vi "HFRR ADV v038.vi"() -> ()   [LabVIEW 2025] (continued)
              }
              frame #2 {
                n259 = local write "Due Write"("VC;0") -> ()
              }
              frame #3 {
                n260 = Wait (ms)(milliseconds to wait=u32 2000) -> ()  [unwired: 1 out]
              }
              frame #4 {
                w347 = T19."Enabled" ("Disabled")
                (unwired) T26."Imaging" ("Main Dashboard Buttons")
                w348 = "" ("FILE")
                n261 = local write "Main Tab"(T2."Adv Scar" ("Main Tab")) -> ()
                n262 = local write "measured_stroke"(0.0 ("measured_stroke")) -> ()
                n263 = local write "Main Dashboard Buttons"(T1."Imaging" ("Main Dashboard Buttons")) -> ()
                n264 = property on="RUN" class="Bool (strict)"("Visible"=TRUE) -> ()  [unwired: 2 in, 2 out]
                n265 = local write "Due Write"("VC;0") -> ()
                n266 = local write "Humidity"(TRUE ("Humidity")) -> ()
                n267 = local write "TEST FILE NAM,E SAVED"(FALSE ("TEST FILE NAM,E SAVED")) -> ()
                n268 = local write "Fuel Discription :"(w348) -> ()
                n269 = local write "Batch Ref Num :"(w348) -> ()
                n270 = local write "Remarks :"(w348) -> ()
                n271 = local write "FILE"(w348) -> ()
                n272 = property on="FRICVALZ 2" class="Bool (strict)"("DisabledEnum"=w347) -> ()  [unwired: 2 in, 2 out]
                n273 = property on="FRICVALZ 4" class="Bool (strict)"("DisabledEnum"=w347) -> ()  [unwired: 2 in, 2 out]
                n274 = property on="FRICVALZ 3" class="Bool (strict)"("DisabledEnum"=w347) -> ()  [unwired: 2 in, 2 out]
              }
            }
          }
          frame True {
            n275 = stacked-sequence {
              frame #0 {
                n276 = local write "Due Write"("DAC;200") -> ()
              }
              frame #1 {
                n277 = Wait (ms)(milliseconds to wait=u32 1500) -> ()  [unwired: 1 out]
              }
              frame #2 {
                n278 = local write "Due Write"("DAC;200") -> ()
              }
              frame #3 {
                n279 = Wait (ms)(milliseconds to wait=u32 1000) -> ()  [unwired: 1 out]
              }
              frame #4 {
                n280 = local write "Due Write"("VC;1") -> ()
              }
              frame #5 {
                n281 = Wait (ms)(milliseconds to wait=u32 2000) -> ()  [unwired: 1 out]
              }
              frame #6 {
                n282 = local write "Due Write"("VC;1") -> ()
              }
              frame #7 {
                n283 = Wait (ms)(milliseconds to wait=u32 2000) -> ()  [unwired: 1 out]
              }
              frame #8 {
                w359 = T19."Disabled" ("Disabled")
                n284 = property on="RUN" class="Bool (strict)"("Visible"=FALSE) -> ()  [unwired: 2 in, 2 out]
                n285 = property on="FRICVALZ 2" class="Bool (strict)"("DisabledEnum"=w359) -> ()  [unwired: 2 in, 2 out]
                n286 = property on="FRICVALZ 4" class="Bool (strict)"("DisabledEnum"=w359) -> ()  [unwired: 2 in, 2 out]
                n287 = property on="FRICVALZ 3" class="Bool (strict)"("DisabledEnum"=w359) -> ()  [unwired: 2 in, 2 out]
                "START TEMP" <- TRUE
              }
            }
          }
        }
      }
      event "FILE", "USERNAME", "USER ID": Mouse Enter {
        n288 = event-data() -> ()  [unwired: 1 in, 4 out]
        n289 = dll-call lib="kernel32.dll" fn="Wow64DisableWow64FsRedirection"("OldValue"=0) -> (error out=w366:errorcluster, "OldValue"=w364:i32)  [unwired: 4 in, 1 out]
        n290 = call <vilib>:"System Exec.vi"("run minimized? (F)"=TRUE, "error in (no error)"=w366, "command line"="C:\\Program Files\\Common Files\\Microsoft Shared\\Ink\\TabTip.exe") -> ("error out"=w365:errorcluster)  [unwired: 5 in, 3 out]
        n291 = dll-call lib="kernel32.dll" fn="Wow64EnableWow64FsRedirection"(error in=w365, "OldValue"=w364) -> ()  [unwired: 4 in, 2 out]
      }
      event "EDIT": Value Change {
        n292 = event-data() -> ()  [unwired: 1 in, 6 out]
        n293 = local read "EDIT"() -> (w367:bool)
        n294 = case shown="False" w367 {
          frame False {
            n295 = control-ref of="This VI"() -> (w384:refnum<vi>)
            n296 = property class="VI"(reference=w384) -> (reference out=w375:refnum<vi>, error out=w379:errorcluster, "Panel"=w383:refnum<vi>)  [unwired: 1 in]
            n297 = property class="Pnl"(reference=w383, error in=w379) -> (reference out=w377:refnum<vi>, error out=w380:errorcluster, "Panes[]"=w382:refnum<vi>[])
            n298 = for {
              tunnel: w382 -> [w390] mode=indexing
              tunnel: T24."Always Off" ("Horizontal Scrollbar Visibility") -> [w389]
              tunnel: w380 -> [w386]
              tunnel: [w385] -> w378
              n299 = property class="Pane"(reference=w390, error in=w386, "HorizScrollbarVisibility"=w389) -> (reference out=w387:refnum<vi>, error out=w388:errorcluster)
              n300 = Close Reference(reference=w387, error in (no error)=w388) -> (error out=w385:errorcluster)
            }
            n301 = Close Reference(reference=w377, error in (no error)=w378) -> (error out=w376:errorcluster)
            n302 = Close Reference(reference=w375, error in (no error)=w376) -> (error out=w370:errorcluster)
            "error out 7" <- w370
            n303 = call <vilib>:"Clear Errors.vi"("error in (no error)"=w370) -> ("error out"=w369:errorcluster)  [unwired: 5 in, 1 out]
            n304 = local write "Service Password enable"(FALSE ("Service Password enable")) -> ()
            n305 = call <userlib>:"Fit VI window to Largest Dec.vi"("error in (no error)"=w369, "border spacing (2 px)"=1) -> ("error out"=w374:errorcluster, "dup VI Ref"=w372:refnum<vi>)  [unwired: 4 in]
            n306 = invoke on="Invoke Node" class="VI" method="FP.Run-Time Position.Maximized"(reference=w372, error in=w374) -> (error out=w373:errorcluster)  [unwired: 2 in, 3 out]
            n307 = call <vilib>:"Clear Errors.vi"("error in (no error)"=w373) -> ()  [unwired: 5 in, 2 out]
          }
          frame True {
          }
        }
      }
      event "Heater Button": Value Change {
        n308 = event-data() -> ()  [unwired: 1 in, 6 out]
        n309 = local read "Heater Button"() -> (w391:bool)
        n310 = case shown="True" w391 {
          frame True {
            n311 = stacked-sequence {
              frame #0 {
                n312 = Wait (ms)(milliseconds to wait=u32 1500) -> ()  [unwired: 1 out]
              }
              frame #1 {
                n313 = local read "Set Temp"() -> (w393:dbl)
                n314 = Number To Fractional String(number=w393, precision (6)=i16 2) -> (F-format string=w396:string)  [unwired: 2 in]
                n315 = Concatenate Strings("ST;" ("Command"), w396) -> (w395:string)
                n316 = local write "Due Write"(w395) -> ()
              }
              frame #2 {
                n317 = Wait (ms)(milliseconds to wait=u32 1500) -> ()  [unwired: 1 out]
              }
              frame #3 {
                n318 = local write "Due Write"("HE;1" ("Command")) -> ()
              }
              frame #4 {
                n319 = Wait (ms)(milliseconds to wait=u32 1500) -> ()  [unwired: 1 out]
              }
              frame #5 {
                n320 = stacked-sequence {
                  frame #0 {
                    n321 = Wait (ms)(milliseconds to wait=u32 1500) -> ()  [unwired: 1 out]
                  }
                  frame #1 {
                    n322 = local read "Set Temp"() -> (w402:dbl)
                    n323 = Number To Fractional String(number=w402, precision (6)=i16 2) -> (F-format string=w405:string)  [unwired: 2 in]
                    n324 = Concatenate Strings("ST;" ("Command"), w405) -> (w404:string)
                    n325 = local write "Due Write"(w404) -> ()
                  }
                  frame #2 {
                    n326 = Wait (ms)(milliseconds to wait=u32 1500) -> ()  [unwired: 1 out]
                  }
                  frame #3 {
                    n327 = local write "Due Write"("HE;1" ("Command")) -> ()
                  }
                  frame #4 {
                    n328 = Wait (ms)(milliseconds to wait=u32 1500) -> ()  [unwired: 1 out]
                  }
                }
              }
            }
          }
          frame False {
            n329 = stacked-sequence {
              frame #0 {
                n330 = Wait (ms)(milliseconds to wait=u32 1500) -> ()  [unwired: 1 out]
              }
              frame #1 {
                n331 = Concatenate Strings("ST;" ("Command"), "0" ("string")) -> (w412:string)
                n332 = local write "Due Write"(w412) -> ()
              }
              frame #2 {
                n333 = Wait (ms)(milliseconds to wait=u32 1500) -> ()  [unwired: 1 out]
              }
              frame #3 {
                n334 = local write "Due Write"("HE;0" ("Command")) -> ()
              }
              frame #4 {
                n335 = Wait (ms)(milliseconds to wait=u32 1500) -> ()  [unwired: 1 out]
              }
            }
          }
        }
      }
      event "Headen Service Button": Value Change {
        n336 = event-data() -> ()  [unwired: 1 in, 6 out]
        n337 = local read "Headen Service Button"() -> (w417:bool)
        n338 = case shown="True" w417 {
          frame False {
            n339 = property on="Password 3" class="Clust (strict)"("Visible"=FALSE) -> ()  [unwired: 2 in, 2 out]
            n340 = property on="Service Password Log" class="Str"("Visible"=FALSE) -> ()  [unwired: 2 in, 2 out]
          }
          frame True {
            n341 = property on="Password 3" class="Clust (strict)"("Visible"=TRUE) -> ()  [unwired: 2 in, 2 out]
            n342 = property on="Service Password Log" class="Str"("Visible"=TRUE) -> ()  [unwired: 2 in, 2 out]
          }
        }
      }
      event "Password 3.Service Password": Value Change {
        n343 = event-data() -> ()  [unwired: 1 in, 6 out]
        n344 = Unbundle By Name("Password 3") -> ("Service Password"=w424:string)
        n345 = call <vilib>:"Trim Whitespace.vi"("string"=w424) -> ("trimmed string"=w422:string)  [unwired: 1 in]
        n346 = Equal?(x=w422, y="Service@123") -> (x = y?=w423:bool)
        n347 = case shown="False" w423 {
          selector: w423 -> [w427 w429]
          frame False {
            n348 = local write "Service Password enable"(w427) -> ()
            n349 = property on="Service Password Log" class="Str"("Visible"=TRUE) -> ()  [unwired: 2 in, 2 out]
          }
          frame True {
            n350 = property on="Service Password Log" class="Str"("Visible"=FALSE) -> ()  [unwired: 2 in, 2 out]
            "Service Password enable" <- w429
          }
        }
      }
      event "Sign In": Value Change {
        w431 = FALSE ("Visible")
        n351 = event-data() -> ()  [unwired: 1 in, 6 out]
        n352 = property on="About" class="Clust (strict)"("Visible"=w431) -> ()  [unwired: 2 in, 2 out]
        n353 = property on="Password 3" class="Clust (strict)"("Visible"=w431) -> ()  [unwired: 2 in, 2 out]
        n354 = property on="Service Password Log" class="Str"("Visible"=FALSE) -> ()  [unwired: 2 in, 2 out]
      }
      event "Info": Value Change {
        n355 = event-data() -> ()  [unwired: 1 in, 6 out]
        n356 = local read "Info"() -> (w433:bool)
        n357 = case shown="False" w433 {
          frame False {
            n358 = property on="About" class="Clust (strict)"("Visible"=FALSE) -> ()  [unwired: 2 in, 2 out]
          }
          frame True {
            n359 = property on="About" class="Clust (strict)"("Visible"=TRUE) -> ()  [unwired: 2 in, 2 out]
          }
        }
      }
      event "Calibration": Value Change {
        n360 = event-data() -> ()  [unwired: 1 in, 6 out]
        n361 = local read "Calibration"() -> (w437:bool)
        n362 = case shown="False" w437 {
          frame False {
            n363 = property on="Calibration 2" class="TabCtl (strict)"("Visible"=FALSE) -> ()  [unwired: 2 in, 2 out]
            n364 = local write "Cal Password"("" ("Cal Password")) -> ()
          }
          frame True {
            n365 = property on="Calibration 2" class="TabCtl (strict)"("Visible"=TRUE) -> ()  [unwired: 2 in, 2 out]
            n366 = local write "Cal Password"("" ("Cal Password")) -> ()
          }
        }
        n367 = property on="Wrong Password" class="Str"("Visible"=FALSE) -> ()  [unwired: 2 in, 2 out]
      }
      event "Cal Password": Value Change {
        n368 = event-data() -> ()  [unwired: 1 in, 6 out]
        n369 = local read "Cal Password"() -> (w445:string)
        n370 = call <vilib>:"Trim Whitespace.vi"("string"=w445) -> ("trimmed string"=w444:string)  [unwired: 1 in]
        n371 = Equal?(x=w444, y="Cal@321") -> (x = y?=w442:bool)
        n372 = case shown="True" w442 {
          frame False {
            n373 = property on="Wrong Password" class="Str"("Visible"=TRUE) -> ()  [unwired: 2 in, 2 out]
          }
          frame True {
            n374 = property on="Wrong Password" class="Str"("Visible"=FALSE) -> ()  [unwired: 2 in, 2 out]
            n375 = local write "Main Tab"(T2."About" ("Main Tab")) -> ()
            n376 = local write "Cal Password"("" ("Cal Password")) -> ()
            n377 = local write "Main Dashboard Buttons"(T1."About" ("Main Dashboard Buttons")) -> ()
            n378 = property on="Calibration 2" class="TabCtl (strict)"("Visible"=FALSE) -> ()  [unwired: 2 in, 2 out]
            n379 = local write "Calibration"(FALSE ("Calibration")) -> ()
          }
        }
      }
      event "Calibration Selection": Value Change {
        n380 = event-data() -> ()  [unwired: 1 in, 6 out]
        n381 = local read "Calibration Selection"() -> (w454:T8)
        n382 = case shown="\"Stroke Calibration\"" w454 {
          tunnel: [T7."Stroke" ("Main Calibration Tab") T7."Friction" ("Main Calibration Tab") T7."Main" ("Main Calibration Tab") T7."Temperature" ("Main Calibration Tab")] -> w453
          frame "Stroke Calibration" {
          }
          frame "Friction Force Calibration" {
          }
          frame Default {
          }
          frame "Temperature Calibration" {
          }
        }
        n383 = local write "Main Calibration Tab"(w453) -> ()
      }
      event "Back Stroke": Value Change {
        n384 = event-data() -> ()  [unwired: 1 in, 6 out]
        n385 = local write "Main Stroke Tab"(T9."Step 1" ("Main Stroke Tab")) -> ()
        n386 = local write "Main Calibration Tab"(T7."Main" ("Main Calibration Tab")) -> ()
        n387 = local write "Back Stroke"(FALSE ("Back Stroke")) -> ()
      }
      event "Step 2 Back": Value Change {
        n388 = event-data() -> ()  [unwired: 1 in, 6 out]
        n389 = local write "Main Stroke Tab"(T9."Step 1" ("Main Stroke Tab")) -> ()
        n390 = local write "Step 2 Back"(FALSE ("Back Stroke")) -> ()
      }
      event "Step 3 Back": Value Change {
        n391 = event-data() -> ()  [unwired: 1 in, 6 out]
        n392 = local write "Main Stroke Tab"(T9."Step 2" ("Main Stroke Tab")) -> ()
        n393 = local write "Step 3 Back"(FALSE ("Back Stroke")) -> ()
      }
      event "Step 4 Back": Value Change {
        n394 = event-data() -> ()  [unwired: 1 in, 6 out]
        n395 = local write "Main Stroke Tab"(T9."Step 3" ("Main Stroke Tab")) -> ()
        n396 = local write "Step 4 Back"(FALSE ("Back Stroke")) -> ()
      }
      event "Step 5 Back": Value Change {
        n397 = event-data() -> ()  [unwired: 1 in, 6 out]
        n398 = local write "Main Stroke Tab"(T9."Step 4" ("Main Stroke Tab")) -> ()
        n399 = local write "Step 5 Back"(FALSE ("Back Stroke")) -> ()
      }
      event "Step 6 Back": Value Change {
        n400 = event-data() -> ()  [unwired: 1 in, 6 out]
        n401 = local write "Main Stroke Tab"(T9."Step 5" ("Main Stroke Tab")) -> ()
        n402 = local write "Step 6 Back"(FALSE ("Back Stroke")) -> ()
      }
      event "Back Stroke step 7": Value Change {
        n403 = event-data() -> ()  [unwired: 1 in, 6 out]
        n404 = local write "Main Stroke Tab"(T9."Step 5" ("Main Stroke Tab")) -> ()
        n405 = local write "Back Stroke step 7"(FALSE ("Back Stroke")) -> ()
      }
      event "Back Stroke step 8": Value Change {
        n406 = event-data() -> ()  [unwired: 1 in, 6 out]
        n407 = local write "Main Stroke Tab"(T9."Step 7" ("Main Stroke Tab")) -> ()
        n408 = local write "Back Stroke step 8"(FALSE ("Back Stroke")) -> ()
      }
      event "Back Stroke 8": Value Change {
        n409 = event-data() -> ()  [unwired: 1 in, 6 out]
        n410 = local write "MOVE CARRIAGE TO"(0.2 ("MOVE CARRIAGE TO")) -> ()
        n411 = local write "Main Stroke Tab"(T9."Step 1" ("Main Stroke Tab")) -> ()
        n412 = local write "Back Stroke 8"(FALSE ("Back Stroke 8")) -> ()
      }
      event "Continue Stroke": Value Change {
        n413 = event-data() -> ()  [unwired: 1 in, 6 out]
        n414 = local write "Main Stroke Tab"(T9."Step 2" ("Main Stroke Tab")) -> ()
        n415 = local write "Continue Stroke"(FALSE ("Continue Stroke")) -> ()
      }
      event "Continue Stroke step 2": Value Change {
        n416 = event-data() -> ()  [unwired: 1 in, 6 out]
        n417 = local write "Main Stroke Tab"(T9."Step 3" ("Main Stroke Tab")) -> ()
        n418 = local write "Continue Stroke step 2"(FALSE ("Continue Stroke")) -> ()
      }
      event "Continue Stroke step 3": Value Change {
        n419 = event-data() -> ()  [unwired: 1 in, 6 out]
        n420 = local write "Main Stroke Tab"(T9."Step 4" ("Main Stroke Tab")) -> ()
        n421 = local write "Continue Stroke step 3"(FALSE ("Continue Stroke")) -> ()
      }
      event "Continue Stroke step 4": Value Change {
        n422 = event-data() -> ()  [unwired: 1 in, 6 out]
        n423 = local write "Main Stroke Tab"(T9."Step 5" ("Main Stroke Tab")) -> ()
        n424 = local write "Continue Stroke step 4"(FALSE ("Continue Stroke")) -> ()
      }
      event "Continue Stroke step 5": Value Change {
        n425 = event-data() -> ()  [unwired: 1 in, 6 out]
        n426 = local write "Main Stroke Tab"(T9."Step 7" ("Main Stroke Tab")) -> ()
        n427 = local write "Continue Stroke step 5"(FALSE ("Continue Stroke")) -> ()
      }
      event "Continue Stroke step 6": Value Change {
        n428 = event-data() -> ()  [unwired: 1 in, 6 out]
        n429 = local write "Main Stroke Tab"(T9."Step 7" ("Main Stroke Tab")) -> ()
        n430 = local write "Continue Stroke step 6"(FALSE ("Continue Stroke")) -> ()
      }
      event "Continue Stroke step 7": Value Change {
        w493 = FALSE ("0.2mm")
        n431 = event-data() -> ()  [unwired: 1 in, 6 out]
        n432 = local write "0.4 mm"(w493) -> ()
        n433 = local write "0.6 mm"(w493) -> ()
        n434 = local write "1.0 mm"(w493) -> ()
        n435 = local write "1.2 mm"(w493) -> ()
        n436 = local write "0.2 2"(w493) -> ()
        n437 = local write "0.4 2"(w493) -> ()
        n438 = local write "0.6 2"(w493) -> ()
        n439 = local write "0.8 2"(w493) -> ()
        n440 = local write "1.0 2"(w493) -> ()
        n441 = local write "1.2"(w493) -> ()
        n442 = local write "0.2mm"(w493) -> ()
        n443 = local write "0.8mm"(w493) -> ()
        n444 = local write "Main Stroke Tab"(T9."Step 8" ("Main Stroke Tab")) -> ()
        n445 = local write "Continue Stroke step 7"(FALSE ("Continue Stroke")) -> ()
        n446 = local write "Stroke Test Complete"(T10."Test Progress" ("Stroke Test Complete")) -> ()
        "Position Measurment Temp" <- 4.0 ("Position Measurment Temp")
        "Calibration Tare" <- TRUE ("Calibration Tare")
        "MOVE CARRIAGE TO" <- 1.0 ("MOVE CARRIAGE TO")
      }
      event "Continue Stroke step 8": Value Change {
        n447 = event-data() -> ()  [unwired: 1 in, 6 out]
        n448 = local read "LVDT STROKE  Calibration"() -> (w498:dbl)
        n449 = local read "Position Measurment Temp"() -> (w499:dbl)
        n450 = case shown="0, Default" w499 {
          selector: w499 -> [w504 w509 w514 w519 _ w527 w530 w531]
          tunnel: w498 -> [w500 w505 w510 w515 w521 w524 _ _]
          frame 0, Default {
            w502 = TRUE ("0.2mm")
            n451 = Increment(x=w504) -> (x+1=w503:i32)
            n452 = local write "Position Measurment Temp"(w503) -> ()
            n453 = local write "0.2mm"(w502) -> ()
            n454 = local write "0.2 2"(w502) -> ()
            n455 = local write "MOVE CARRIAGE TO"(1.0 ("MOVE CARRIAGE TO")) -> ()
            "Calibration 0.2" <- w500
          }
          frame 1 {
            w507 = TRUE ("0.4 mm")
            n456 = Increment(x=w509) -> (x+1=w508:i32)
            n457 = local write "Calibration 0.4"(w505) -> ()
            n458 = local write "Position Measurment Temp"(w508) -> ()
            n459 = local write "0.4 mm"(w507) -> ()
            n460 = local write "MOVE CARRIAGE TO"(0.6 ("MOVE CARRIAGE TO")) -> ()
            n461 = local write "0.4 2"(w507) -> ()
          }
          frame 2 {
            w512 = TRUE ("0.6 mm")
            n462 = Increment(x=w514) -> (x+1=w513:i32)
            n463 = local write "Calibration 0.6"(w510) -> ()
            n464 = local write "Position Measurment Temp"(w513) -> ()
            n465 = local write "0.6 2"(w512) -> ()
            n466 = local write "0.6 mm"(w512) -> ()
            n467 = local write "MOVE CARRIAGE TO"(0.8 ("MOVE CARRIAGE TO")) -> ()
          }
          frame 3 {
            w516 = TRUE ("0.6 mm")
            n468 = Increment(x=w519) -> (x+1=w518:i32)
            n469 = local write "Position Measurment Temp"(w518) -> ()
            n470 = local write "MOVE CARRIAGE TO"(1.0 ("MOVE CARRIAGE TO")) -> ()
            n471 = local write "0.8mm"(w516) -> ()
            n472 = local write "0.8 2"(w516) -> ()
            "Calibration 0.8" <- w515
          }
          frame 4 {
            w522 = TRUE ("0.6 mm")
            n473 = local write "Position Measurment Temp"(6.0 ("Position Measurment Temp")) -> ()
            n474 = local write "MOVE CARRIAGE TO"(1.0 ("MOVE CARRIAGE TO")) -> ()
            n475 = local write "1.0 mm"(w522) -> ()
            n476 = local write "1.0 2"(w522) -> ()
            "Calibration 1.0" <- w521
          }
          frame 5 {
            w525 = TRUE ("0.6 mm")
            n477 = Increment(x=w527) -> (x+1=w526:i32)
            n478 = local write "Position Measurment Temp"(w526) -> ()
            n479 = local write "1.2 mm"(w525) -> ()
            n480 = local write "1.2"(w525) -> ()
            "Calibration 1.2" <- w524
          }
          frame 6 {
            n481 = Increment(x=w530) -> (x+1=w529:i32)
            n482 = local write "Position Measurment Temp"(w529) -> ()
            n483 = local write "Stroke Test Complete"(T10."Stroke Points Completed" ("Stroke Test Complete")) -> ()
          }
          frame 7 {
            n484 = stacked-sequence {
              tunnel: w531 -> [w532 _ _]
              frame #0 {
                n485 = Increment(x=w532) -> (x+1=w533:i32)
                n486 = local write "Main Stroke Tab"(T9."Step 9" ("Main Stroke Tab")) -> ()
                n487 = local write "Position Measurment Temp"(w533) -> ()
                n488 = Insert Into Array(array=dbl[] [], new element #1=0.2 ("new element/subarray"), new element #2=0.4 ("new element/subarray"), new element #3=0.6 ("new element/subarray"), new element #4=0.8 ("new element/subarray"), new element #5=1.0 ("new element/subarray"), new element #6=1.2 ("new element/subarray")) -> (→"1D stroke":dbl[])  [unwired: 1 in]
                n489 = local read "Calibration 0.2"() -> (w540:dbl)
                n490 = local read "Calibration 0.4"() -> (w539:dbl)
                n491 = local read "Calibration 0.6"() -> (w538:dbl)
                n492 = local read "Calibration 0.8"() -> (w537:dbl)
                n493 = local read "Calibration 1.0"() -> (w536:dbl)
                n494 = local read "Calibration 1.2"() -> (w535:dbl)
                n495 = Insert Into Array(array=dbl[] [], new element #1=w540, new element #2=w539, new element #3=w538, new element #4=w537, new element #5=w536, new element #6=w535) -> (→"Calibrated Voltage Value":dbl[])  [unwired: 1 in]
              }
              frame #1 {
                n496 = local read "calibration values"() -> (w563:dbl[])
                n497 = local read "Calibrated Voltage Value"() -> (w565:dbl[])
                n498 = Index Array(array=w563, index #1=1 ("index"), index #2=3 ("index"), index #3=5 ("index"), index #4=7 ("index"), index #5=9 ("index"), index #6=11 ("index")) -> (element #1=w556:dbl, element #2=w555:dbl, element #3=w554:dbl, element #4=w553:dbl, element #5=w552:dbl, element #6=w551:dbl)
                n499 = local read "1D stroke"() -> (w566:dbl[])
                n500 = for {
                  tunnel: [w575] -> w564 mode=indexing
                  tunnel: w566 -> [w574] mode=indexing
                  tunnel: w565 -> [w573] mode=indexing
                  tunnel: w556 -> [w572]
                  tunnel: w555 -> [w571]
                  tunnel: w554 -> [w570]
                  tunnel: w553 -> [w569]
                  tunnel: w552 -> [w568]
                  tunnel: w551 -> [w567]
                  n501 = formula code="if (stroke == 0.2)\n{\n    if ((voltage >= REF_02 - 0.2) && (voltage <= REF_02 + 0.2))\n        status = 1;\n    else\n        status = 0;\n}\nelse if (stroke == 0.4)\n{\n    if ((voltage >= REF_04 - 0.2) && (voltage <= REF_04 + 0.2))\n        status = 1;\n    else\n        status = 0;\n}\nelse if (stroke == 0.6)\n{\n    if ((voltage >= REF_06 - 0.2) && (voltage <= REF_06 + 0.2))\n        status = 1;\n    else\n        status = 0;\n}\nelse if (stroke == 0.8)\n{\n    if ((voltage >= REF_08 - 0.2) && (voltage <= REF_08 + 0.2))\n        status = 1;\n    else\n        status = 0;\n}\nelse if (stroke == 1.0)\n{\n    if ((voltage >= REF_10 - 0.4) && (voltage <= REF_10 + 0.4))\n        status = 1;\n    else\n        status = 0;\n}\nelse if (stroke == 1.2)\n{\n    if ((voltage >= REF_12 - 0.2) && (voltage <= REF_12 + 0.2))\n        status = 1;\n    else\n        status = 0;\n}\nelse\n{\n    status = 0;\n}"("stroke"=w574, "voltage"=w573, "REF_02"=w572, "REF_04"=w571, "REF_06"=w570, "REF_08"=w569, "REF_10"=w568, "REF_12"=w567) -> ("status"=w575:dbl)
                }
                "Status" <- w564
              }
              frame #2 {
                w582 = 1.0
                n502 = local read "Status"() -> (w589:dbl[])
                n503 = Index Array(array=w589) -> (element #1=w588:dbl, element #2=w587:dbl, element #3=w586:dbl, element #4=w585:dbl, element #5=w584:dbl, element #6=w583:dbl)  [unwired: 6 in]
                n504 = Equal?(x=w587, y=w582) -> (x = y?=w580:bool)
                n505 = Equal?(x=w586, y=w582) -> (x = y?=w579:bool)
                n506 = Equal?(x=w585, y=w582) -> (x = y?=w578:bool)
                n507 = Equal?(x=w584, y=w582) -> (x = y?=w577:bool)
                n508 = Equal?(x=w583, y=w582) -> (x = y?=w576:bool)
                n509 = Equal?(x=w588, y=w582) -> (x = y?=w581:bool)
                n510 = case shown="True" w581 {
                  selector: w581 -> [w600 w601]
                  frame True {
                    n511 = local write "Point 1 - 0.2 mm"(w600) -> ()
                    n512 = property on="Point 1 - 0.2 mm" class="Bool"("Caption.Visible"=w600) -> ()  [unwired: 2 in, 2 out]
                  }
                  frame False {
                    n513 = local write "Point 1 - 0.2 mm"(w601) -> ()
                    n514 = property on="Point 1 - 0.2 mm" class="Bool"("Caption.Visible"=w601) -> ()  [unwired: 2 in, 2 out]
                  }
                }
                n515 = case shown="True" w580 {
                  selector: w580 -> [w598 w599]
                  frame True {
                    n516 = local write "Point 2 - 0.4 mm"(w598) -> ()
                    n517 = property on="Point 2 - 0.4 mm" class="Bool"("Caption.Visible"=w598) -> ()  [unwired: 2 in, 2 out]
                  }
                  frame False {
                    n518 = local write "Point 2 - 0.4 mm"(w599) -> ()
                    n519 = property on="Point 2 - 0.4 mm" class="Bool"("Caption.Visible"=w599) -> ()  [unwired: 2 in, 2 out]
                  }
                }
                n520 = case shown="True" w577 {
                  selector: w577 -> [w592 w593]
                  frame True {
                    n521 = local write "Point 5 - 1.0 mm"(w592) -> ()
                    n522 = property on="Point 5 - 1.0 mm" class="Bool"("Caption.Visible"=w592) -> ()  [unwired: 2 in, 2 out]
                  }
                  frame False {
                    n523 = local write "Point 5 - 1.0 mm"(w593) -> ()
                    n524 = property on="Point 5 - 1.0 mm" class="Bool"("Caption.Visible"=w593) -> ()  [unwired: 2 in, 2 out]
                  }
                }
                n525 = case shown="True" w579 {
                  selector: w579 -> [w596 w597]
                  frame True {
                    n526 = local write "Point 3 - 0.6 mm"(w596) -> ()
                    n527 = property on="Point 3 - 0.6 mm" class="Bool"("Caption.Visible"=w596) -> ()  [unwired: 2 in, 2 out]
                  }
                  frame False {
                    n528 = local write "Point 3 - 0.6 mm"(w597) -> ()
                    n529 = property on="Point 3 - 0.6 mm" class="Bool"("Caption.Visible"=w597) -> ()  [unwired: 2 in, 2 out]
                  }
                }
                n530 = case shown="True" w578 {
                  selector: w578 -> [w594 w595]
                  frame True {
                    n531 = local write "Point 4 - 0.8 mm"(w594) -> ()
                    n532 = property on="Point 4 - 0.8 mm" class="Bool"("Caption.Visible"=w594) -> ()  [unwired: 2 in, 2 out]
                  }
                  frame False {
                    n533 = local write "Point 4 - 0.8 mm"(w595) -> ()
                    n534 = property on="Point 4 - 0.8 mm" class="Bool"("Caption.Visible"=w595) -> ()  [unwired: 2 in, 2 out]
                  }
                }
                n535 = case shown="True" w576 {
                  selector: w576 -> [w590 w591]
                  frame True {
                    n536 = local write "Point 6 - 1.2 mm"(w590) -> ()
                    n537 = property on="Point 6 - 1.2 mm" class="Bool"("Caption.Visible"=w590) -> ()  [unwired: 2 in, 2 out]
                  }
                  frame False {
                    n538 = local write "Point 6 - 1.2 mm"(w591) -> ()
                    n539 = property on="Point 6 - 1.2 mm" class="Bool"("Caption.Visible"=w591) -> ()  [unwired: 2 in, 2 out]
                  }
                }
              }
            }
          }
        }
      }
      event "TEMPERATURE STEP Back 1", "TEMPERATURE STEP Back air Temp": Value Change {
        n540 = event-data() -> ()  [unwired: 1 in, 6 out]
        n541 = stacked-sequence {
          frame #0 {
            n542 = local write "Main Calibration Tab"(T7."Main" ("Main Calibration Tab")) -> ()
          }
          frame #1 {
            n543 = Wait (ms)(milliseconds to wait=u32 1000) -> ()  [unwired: 1 out]
          }
          frame #2 {
            n544 = local write "Due Write"("CAL;END" ("Command")) -> ()
          }
          frame #3 {
            n545 = Wait (ms)(milliseconds to wait=u32 2000) -> ()  [unwired: 1 out]
          }
          frame #4 {
            n546 = local write "Due Write"("CAL;END" ("Command")) -> ()
          }
        }
      }
      event "Temperature Continue Step 1": Value Change {
        n547 = event-data() -> ()  [unwired: 1 in, 6 out]
        n548 = stacked-sequence {
          frame #0 {
            n549 = Wait (ms)(milliseconds to wait=u32 1500) -> ()  [unwired: 1 out]
          }
          frame #1 {
            n550 = local write "Due Write"("CAL;START" ("Command")) -> ()
          }
          frame #2 {
            n551 = Wait (ms)(milliseconds to wait=u32 1500) -> ()  [unwired: 1 out]
          }
          frame #3 {
            n552 = local write "Due Write"("CAL;START" ("Command")) -> ()
          }
          frame #4 {
            n553 = Wait (ms)(milliseconds to wait=u32 2000) -> ()  [unwired: 1 out]
          }
          frame #5 {
          }
          frame #6 {
            n554 = Wait (ms)(milliseconds to wait=u32 2000) -> ()  [unwired: 1 out]
          }
          frame #7 {
            # "CAL;A1;<true_T>"
            n555 = local write "Due Write"("CAL;A1;0" ("Command")) -> ()
          }
          frame #8 {
            n556 = local write "Tab Control 4"(T12."Step 2" ("Tab Control 4")) -> ()
          }
        }
      }
      event "Temperature Continue Step air Step 1": Value Change {
        n557 = event-data() -> ()  [unwired: 1 in, 6 out]
        n558 = stacked-sequence {
          frame #0 {
            n559 = Wait (ms)(milliseconds to wait=u32 1500) -> ()  [unwired: 1 out]
          }
          frame #1 {
            n560 = local write "Due Write"("CAL;START" ("Command")) -> ()
          }
          frame #2 {
            n561 = Wait (ms)(milliseconds to wait=u32 1500) -> ()  [unwired: 1 out]
          }
          frame #3 {
            n562 = local write "Due Write"("CAL;START" ("Command")) -> ()
          }
          frame #4 {
            n563 = Wait (ms)(milliseconds to wait=u32 2000) -> ()  [unwired: 1 out]
          }
          frame #5 {
          }
          frame #6 {
            n564 = Wait (ms)(milliseconds to wait=u32 2000) -> ()  [unwired: 1 out]
          }
          frame #7 {
            # "CAL;A1;<true_T>"
            n565 = local write "Due Write"("CAL;A1;0" ("Command")) -> ()
          }
          frame #8 {
            n566 = local write "Tab Control 4"(T12."Air Step 2" ("Tab Control 4")) -> ()
          }
        }
      }
      event "Temperature Selection": Value Change {
        n567 = event-data() -> ()  [unwired: 1 in, 6 out]
        n568 = local read "Temperature Selection"() -> (w623:T13)
        n569 = case shown="\"Sample Temperature\"" w623 {
          frame "Air Temperature" {
            n570 = local write "Tab Control 4"(T12."Air Step 1" ("Tab Control 4")) -> ()
          }
          frame "Sample Temperature" {
            n571 = local write "Tab Control 4"(T12."Step 1" ("Tab Control 4")) -> ()
          }
          frame "Default", Default {
          }
        }
      }
      event "Temperature Continue Step 2": Value Change {
        n572 = event-data() -> ()  [unwired: 1 in, 6 out]
        n573 = stacked-sequence {
          frame #0 {
            n574 = stacked-sequence {
              frame #0 {
                n575 = Wait (ms)(milliseconds to wait=u32 1500) -> ()  [unwired: 1 out]
              }
              frame #1 {
                # "CAL;A1;<true_T>"
                n576 = local read "Sensor value"() -> (→"Sample 0deg temp":dbl)
                n577 = local write "Due Write"("CAL;A1;0" ("Command")) -> ()
              }
              frame #2 {
                n578 = Wait (ms)(milliseconds to wait=u32 1500) -> ()  [unwired: 1 out]
              }
              frame #3 {
                # "CAL;A1;<true_T>"
                n579 = local write "Due Write"("CAL;A1;0" ("Command")) -> ()
              }
              frame #4 {
              }
            }
          }
          frame #1 {
            n580 = local write "Tab Control 4"(T12."Step 3" ("Tab Control 4")) -> ()
          }
        }
      }
      event "Temperature Continue Air Step 2": Value Change {
        n581 = event-data() -> ()  [unwired: 1 in, 6 out]
        n582 = stacked-sequence {
          frame #0 {
            n583 = stacked-sequence {
              frame #0 {
                n584 = Wait (ms)(milliseconds to wait=u32 1000) -> ()  [unwired: 1 out]
              }
              frame #1 {
                # "CAL;A1;<true_T>"
                n585 = local write "Due Write"("CAL;A1;0" ("Command")) -> ()
              }
              frame #2 {
                n586 = Wait (ms)(milliseconds to wait=u32 1000) -> ()  [unwired: 1 out]
              }
              frame #3 {
                # "CAL;A1;<true_T>"
                n587 = local write "Due Write"("CAL;A1;0" ("Command")) -> ()
              }
              frame #4 {
                n588 = local read "Sensor value"() -> (→"Air 0deg temp":dbl)
              }
            }
          }
          frame #1 {
            n589 = local write "Tab Control 4"(T12."Air Step 3" ("Tab Control 4")) -> ()
          }
        }
      }
      event "Temperature Continue Step 3": Value Change {
        n590 = event-data() -> ()  [unwired: 1 in, 6 out]
        n591 = stacked-sequence {
          frame #0 {
            n592 = stacked-sequence {
              frame #0 {
                n593 = Wait (ms)(milliseconds to wait=u32 1500) -> ()  [unwired: 1 out]
              }
              frame #1 {
              }
              frame #2 {
              }
              frame #3 {
                # "CAL;A1;<true_T>"
                n594 = local write "Due Write"("CAL;A1;60" ("Command")) -> ()
              }
              frame #4 {
                n595 = Wait (ms)(milliseconds to wait=u32 1000) -> ()  [unwired: 1 out]
              }
              frame #5 {
                # "CAL;A1;<true_T>"
                n596 = local read "Sensor value"() -> (→"Sample 60deg temp":dbl)
                n597 = local write "Due Write"("CAL;A1;60" ("Command")) -> ()
              }
            }
          }
          frame #1 {
            n598 = local read "Sample 0deg temp"() -> (w652:dbl)
            n599 = local read "Sample 60deg temp"() -> (w651:dbl)
            n600 = Add(x=w651, y="Temperature diff") -> (x+y=w649:dbl)
            n601 = Subtract(x=w651, y="Temperature diff") -> (x-y=w648:dbl)
            n602 = Add(x=w652, y="Temperature diff") -> (x+y=w647:dbl)
            n603 = Subtract(x=w652, y="Temperature diff") -> (x-y=w646:dbl)
            n604 = In Range and Coerce(upper limit=w649, x=w651, lower limit=w648) -> (In Range?=w645:bool)  [unwired: 1 out]
            n605 = In Range and Coerce(upper limit=w647, x=w652, lower limit=w646) -> (In Range?=w644:bool)  [unwired: 1 out]
            n606 = And(x=w645, y=w644) -> (x .and. y?=w643:bool)
            n607 = case shown="True" w643 {
              frame False {
                n608 = property on="Accept & Save sample Temperature step 4" class="Bool (strict)"("DisabledEnum"=T19."Disabled" ("Disabled")) -> ()  [unwired: 2 in, 2 out]
                n609 = local write "Sample Temperature Calibration  2"(enum32{"True", "Fail"}."Fail" ("Sample Temperature Calibration  2")) -> ()
              }
              frame True {
                n610 = property on="Accept & Save sample Temperature step 4" class="Bool (strict)"("DisabledEnum"=T19."Enabled" ("Disabled")) -> ()  [unwired: 2 in, 2 out]
                n611 = local write "Sample Temperature Calibration  2"(enum32{"True", "Fail"}."True" ("Sample Temperature Calibration  2")) -> ()
              }
            }
          }
          frame #2 {
          }
          frame #3 {
          }
          frame #4 {
          }
          frame #5 {
          }
          frame #6 {
            # "CAL;END"
          }
          frame #7 {
          }
          frame #8 {
            # "CAL;END"
          }
          frame #9 {
            n612 = local write "Tab Control 4"(T12."Step 4" ("Tab Control 4")) -> ()
          }
        }
      }
      event "Accept & Save sample Temperature step 4": Value Change {
        n613 = event-data() -> ()  [unwired: 1 in, 6 out]
        n614 = stacked-sequence {
          frame #0 {
            n615 = local write "Due Write"("CAL;SAVE" ("Command")) -> ()
          }
          frame #1 {
            n616 = Wait (ms)(milliseconds to wait=u32 1000) -> ()  [unwired: 1 out]
          }
          frame #2 {
            n617 = local write "Due Write"("CAL;SAVE" ("Command")) -> ()
          }
          frame #3 {
            n618 = Wait (ms)(milliseconds to wait=u32 1000) -> ()  [unwired: 1 out]
          }
          frame #4 {
            n619 = local write "Due Write"("CAL;END" ("Command")) -> ()
          }
          frame #5 {
            n620 = Wait (ms)(milliseconds to wait=u32 1000) -> ()  [unwired: 1 out]
          }
          frame #6 {
            n621 = local write "Due Write"("CAL;END" ("Command")) -> ()
            n622 = local write "Tab Control 4"(T12."Main" ("Tab Control 4")) -> ()
            n623 = local write "Main Calibration Tab"(T7."Temperature" ("Main Calibration Tab")) -> ()
          }
        }
      }
      event "Accept & Save Air Temperature step 4": Value Change {
        n624 = event-data() -> ()  [unwired: 1 in, 6 out]
        n625 = stacked-sequence {
          frame #0 {
            n626 = local write "Due Write"("CAL;SAVE" ("Command")) -> ()
          }
          frame #1 {
            n627 = Wait (ms)(milliseconds to wait=u32 1000) -> ()  [unwired: 1 out]
          }
          frame #2 {
            n628 = local write "Due Write"("CAL;SAVE" ("Command")) -> ()
          }
          frame #3 {
            n629 = Wait (ms)(milliseconds to wait=u32 1000) -> ()  [unwired: 1 out]
          }
          frame #4 {
            n630 = local write "Due Write"("CAL;END" ("Command")) -> ()
          }
          frame #5 {
            n631 = Wait (ms)(milliseconds to wait=u32 1000) -> ()  [unwired: 1 out]
          }
          frame #6 {
            n632 = local write "Due Write"("CAL;END" ("Command")) -> ()
            n633 = local write "Tab Control 4"(T12."Main" ("Tab Control 4")) -> ()
            n634 = local write "Main Calibration Tab"(T7."Temperature" ("Main Calibration Tab")) -> ()
          }
        }
      }
      event "Temperature Continue Step 6": Value Change {
        n635 = event-data() -> ()  [unwired: 1 in, 6 out]
        n636 = stacked-sequence {
          frame #0 {
            n637 = stacked-sequence {
              frame #0 {
                n638 = Wait (ms)(milliseconds to wait=u32 1000) -> ()  [unwired: 1 out]
              }
              frame #1 {
              }
              frame #2 {
              }
              frame #3 {
                # "CAL;A1;<true_T>"
                n639 = local write "Due Write"("CAL;A1;60" ("Command")) -> ()
              }
              frame #4 {
                n640 = Wait (ms)(milliseconds to wait=u32 1000) -> ()  [unwired: 1 out]
              }
              frame #5 {
                # "CAL;A1;<true_T>"
                n641 = local write "Due Write"("CAL;A1;60" ("Command")) -> ()
              }
            }
          }
          frame #1 {
            n642 = local read "Sensor value"() -> (→"Air 60deg temp":dbl)
          }
          frame #2 {
          }
          frame #3 {
          }
          frame #4 {
          }
          frame #5 {
          }
          frame #6 {
            # "CAL;END"
          }
          frame #7 {
            n643 = local read "Temperature diff"() -> (w683:dbl)
            n644 = local read "Air 60deg temp"() -> (w682:dbl)
            n645 = local read "Air 0deg temp"() -> (w681:dbl)
            n646 = Add(x=w682, y=w683) -> (x+y=w690:dbl)
            n647 = Subtract(x=w682, y=w683) -> (x-y=w689:dbl)
            n648 = Add(x=w681, y=w683) -> (x+y=w688:dbl)
            n649 = Subtract(x=w681, y=w683) -> (x-y=w687:dbl)
            n650 = In Range and Coerce(upper limit=w690, x=w682, lower limit=w689) -> (In Range?=w686:bool)  [unwired: 1 out]
            n651 = In Range and Coerce(upper limit=w688, x=w681, lower limit=w687) -> (In Range?=w685:bool)  [unwired: 1 out]
            n652 = And(x=w686, y=w685) -> (x .and. y?=w684:bool)
            n653 = case shown="True" w684 {
              frame False {
                n654 = property on="Accept & Save Air Temperature step 4" class="Bool (strict)"("DisabledEnum"=T19."Disabled" ("Disabled")) -> ()  [unwired: 2 in, 2 out]
                n655 = local write "Sample Temperature Calibration"(enum32{"True", "Fail"}."Fail" ("Sample Temperature Calibration  2")) -> ()
              }
              frame True {
                n656 = local write "Sample Temperature Calibration"(enum32{"True", "Fail"}."True" ("Sample Temperature Calibration  2")) -> ()
                n657 = property on="Accept & Save Air Temperature step 4" class="Bool (strict)"("DisabledEnum"=T19."Enabled" ("Disabled")) -> ()  [unwired: 2 in, 2 out]
              }
            }
          }
          frame #8 {
            # "CAL;END"
          }
          frame #9 {
            n658 = local write "Tab Control 4"(T12."Air Step 4" ("Tab Control 4")) -> ()
          }
        }
      }
      event "Back Stroke step main temperature": Value Change {
        n659 = event-data() -> ()  [unwired: 1 in, 6 out]
        n660 = stacked-sequence {
          frame #0 {
            n661 = Wait (ms)(milliseconds to wait=u32 1000) -> ()  [unwired: 1 out]
          }
          frame #1 {
            # "CAL;END"
            n662 = local write "Due Write"("CAL;END" ("Command")) -> ()
          }
          frame #2 {
            n663 = Wait (ms)(milliseconds to wait=u32 1000) -> ()  [unwired: 1 out]
          }
          frame #3 {
            # "CAL;END"
            n664 = local write "Due Write"("CAL;END" ("Command")) -> ()
          }
          frame #4 {
            n665 = local write "Main Calibration Tab"(T7."Main" ("Main Calibration Tab")) -> ()
            n666 = local write "Tab Control 4"(T12."Main" ("Tab Control 4")) -> ()
          }
        }
      }
      event "TEMPERATURE STEP  Back 4", "TEMPERATURE STEP 1 Back 3", "TEMPERATURE STEP  Back 3", "TEMPERATURE STEP 1 Back 2", "Back Air TEMPERATURE Step 4", "Back SAMPLE TEMPERATURE Step 4": Value Change {
        # "Back Stroke step main temperature"
        n667 = event-data() -> ()  [unwired: 1 in, 6 out]
        n668 = stacked-sequence {
          frame #0 {
            n669 = Wait (ms)(milliseconds to wait=u32 1000) -> ()  [unwired: 1 out]
          }
          frame #1 {
            # "CAL;END"
            n670 = local write "Due Write"("CAL;END" ("Command")) -> ()
          }
          frame #2 {
            n671 = Wait (ms)(milliseconds to wait=u32 1000) -> ()  [unwired: 1 out]
          }
          frame #3 {
            # "CAL;END"
            n672 = local write "Due Write"("CAL;END" ("Command")) -> ()
          }
          frame #4 {
            # "TEMPERATURE STEP  Back 4"
            n673 = local write "Main Calibration Tab"(T7."Temperature" ("Main Calibration Tab")) -> ()
            n674 = local write "Tab Control 4"(T12."Main" ("Tab Control 4")) -> ()
          }
        }
      }
      event "FF BACK", "FF BACK 2", "FF BACK 3", "FF BACK 4", "FF BACK 5", "FF BACK 6": Value Change {
        n675 = event-data() -> ()  [unwired: 1 in, 6 out]
        n676 = stacked-sequence {
          frame #0 {
            n677 = Wait (ms)(milliseconds to wait=u32 1500) -> ()  [unwired: 1 out]
          }
          frame #1 {
            n678 = local write "Due Write"("VC;0") -> ()
          }
          frame #2 {
            n679 = Wait (ms)(milliseconds to wait=u32 1500) -> ()  [unwired: 1 out]
          }
          frame #3 {
            n680 = local write "Due Write"("VC;0") -> ()
          }
          frame #4 {
            w712 = FALSE
            n681 = local write "FF BACK 2"(w712) -> ()
            n682 = local write "FF BACK 3"(w712) -> ()
            n683 = local write "FF BACK 4"(w712) -> ()
            n684 = local write "FF BACK 5"(w712) -> ()
            n685 = local write "FF BACK 6"(w712) -> ()
            n686 = local write "FF BACK"(w712) -> ()
          }
          frame #5 {
            n687 = local write "Friction Force Tab"(T25."Page 1" ("Friction Force Tab")) -> ()
            n688 = local write "Main Calibration Tab"(T7."Main" ("Main Calibration Tab")) -> ()
          }
        }
      }
      event "FF CONTINUE": Value Change {
        n689 = event-data() -> ()  [unwired: 1 in, 6 out]
        n690 = local write "FF CONTINUE"(FALSE ("FF CONTINUE")) -> ()
        n691 = local write "Friction Force Tab"(T25."Page 2" ("Friction Force Tab")) -> ()
      }
      event "FF CONTINUE 2": Value Change {
        n692 = event-data() -> ()  [unwired: 1 in, 6 out]
        n693 = local write "FF CONTINUE 2"(FALSE ("FF CONTINUE")) -> ()
        n694 = local write "Friction Force Tab"(T25."Page 3" ("Friction Force Tab")) -> ()
      }
      event "FF CONTINUE 3": Value Change {
        n695 = event-data() -> ()  [unwired: 1 in, 6 out]
        n696 = local write "FF CONTINUE 3"(FALSE ("FF CONTINUE")) -> ()
        n697 = local write "Friction Force Tab"(T25."Page 4" ("Friction Force Tab")) -> ()
      }
      event "FF CONTINUE 4": Value Change {
        n698 = event-data() -> ()  [unwired: 1 in, 6 out]
        n699 = local write "FF CONTINUE 4"(FALSE ("FF CONTINUE")) -> ()
        n700 = local write "Friction Force Tab"(T25."Page 5" ("Friction Force Tab")) -> ()
      }
      event "FF CONTINUE 5": Value Change {
        n701 = event-data() -> ()  [unwired: 1 in, 6 out]
        n702 = local write "FF CONTINUE 5"(FALSE ("FF CONTINUE")) -> ()
        n703 = local write "Friction Force Tab"(T25."Page 6" ("Friction Force Tab")) -> ()
      }
      event "Quit": Value Change {
        n704 = event-data() -> ()  [unwired: 1 in, 6 out]
      }
    }
    n705 = Wait (ms)(milliseconds to wait=u32 100) -> ()  [unwired: 1 out]
  }
  n706 = while {
    stop <- w735 stop-if-true
    n707 = local read "Ambient Temperature"() -> (w733:dbl)
    n708 = local read "Sample Temperature"() -> (w732:dbl)
    n709 = Wait (ms)(milliseconds to wait=u32 200) -> ()  [unwired: 1 out]
    n710 = local write "Temperature — Live (Set A: 0 °C)"(w733) -> ()
    n711 = local write "Temperature — Live (Set A: 60 °C)"(w733) -> ()
    n712 = local write "Sensor value"(w733) -> ()
    n713 = local write "Sensor value"(w733) -> ()
    n714 = local write "Sensor value"(w732) -> ()
    n715 = local write "Sensor value"(w732) -> ()
    n716 = local write "Temperature — Live (Set A: 60 °C)"(w732) -> ()
    n717 = local write "Temperature — Live (Set A: 0 °C)"(w732) -> ()
    n718 = case shown="True" "Save Button" {
      selector: "Save Button" -> [_ w762]
      frame False {
      }
      frame True {
        n719 = Not(x=w762) -> (.not. x?=w761:bool)
        n720 = local read "milliseconds to wait"() -> (w794:u32)
        n721 = local read "max_step_change"() -> (w799:dbl)
        n722 = local read "max_amplitude"() -> (w800:dbl)
        n723 = local read "min_amplitude"() -> (w801:dbl)
        n724 = local read "PIEZO_CAL_FACTOR"() -> (w805:dbl)
        n725 = local write "Save Button"(w761) -> ()
        n726 = local read "startup_cmd"() -> (w802:dbl)
        n727 = local read "NORMAL_FORCE"() -> (w806:dbl)
        n728 = local read "ADC_Resolution"() -> (w804:dbl)
        n729 = local read "calibration values"() -> (w809:dbl[])
        n730 = local read "kp"() -> (w796:dbl)
        n731 = local read "kd"() -> (w798:dbl)
        n732 = local read "dt"() -> (w795:dbl)
        n733 = local read "ki"() -> (w797:dbl)
        n734 = local read "STROKE FILTER"() -> (w807:i32)
        n735 = local read "Add up Stroke"() -> (w808:dbl)
        n736 = local read "VREF"() -> (w803:dbl)
        n737 = Insert Into Array(array=dbl[] [], new element #1=w794, new element #2=w795, new element #3=w796, new element #4=w797, new element #5=w798, new element #6=w799, new element #7=w800, new element #8=w801, new element #9=w802) -> (w810:dbl[])  [unwired: 1 in]
        n738 = Insert Into Array(array=dbl[] [], new element #1=w803, new element #2=w804, new element #3=w805, new element #4=w806) -> (w811:dbl[])  [unwired: 1 in]
        n739 = Array To Spreadsheet String(delimiter (Tab)=";", array=w809, 3:"" ("format string")) -> (spreadsheet string=w813:string)
        n740 = Insert Into Array(array=dbl[] [], new element #1=w807, new element #2=w808) -> (w812:dbl[])  [unwired: 1 in]
        n741 = call "Write Config.vi"("Stroke Calibration"=w813, "STROKE PARAMETERS"=w812, "ADC PARAMETERS"=w811, "PID  PARAMETERS"=w810) -> ("error out"=w792:errorcluster)  [unwired: 7 in]
        n742 = call "Stall Data Flow.vim"("value in"=w792, "milliseconds to wait"=u32 2000) -> ("value out"=w793:errorcluster)  [unwired: 1 out]
        n743 = call "Read Config.vi"("error in (no error)"=w793) -> ("STROKE PARAMETERS"=w790:dbl[], "ADC PARAMETERS"=w789:dbl[], "PID  PARAMETERS"=w788:dbl[], "Stroke Calibration"=w791:string)  [unwired: 5 in, 2 out]
        n744 = Index Array(array=w788) -> (element #1=w786:dbl, element #2=w785:dbl, element #3=w784:dbl, element #4=w783:dbl, element #5=w782:dbl, element #6=w781:dbl, element #7=w780:dbl, element #8=w779:dbl, element #9=w778:dbl)  [unwired: 9 in]
        n745 = Index Array(array=w789) -> (element #1=w777:dbl, element #2=w776:dbl, element #3=w775:dbl, element #4=w774:dbl)  [unwired: 4 in]
        n746 = Index Array(array=w790) -> (element #1=w773:dbl, element #2=w772:dbl)  [unwired: 2 in]
        n747 = Spreadsheet String To Array(delimiter (Tab)=";", format string="", spreadsheet string=w791, array type (2D Dbl)=dbl[] []) -> (array=w787:dbl[])
        n748 = local write "VREF"(w777) -> ()
        n749 = local write "ADC_Resolution"(w776) -> ()
        n750 = local write "PIEZO_CAL_FACTOR"(w775) -> ()
        n751 = local write "NORMAL_FORCE"(w774) -> ()
        n752 = local write "STROKE FILTER"(w773) -> ()
        n753 = local write "Add up Stroke"(w772) -> ()
        n754 = local write "calibration values"(w787) -> ()
        n755 = local write "milliseconds to wait"(w786) -> ()
        n756 = local write "dt"(w785) -> ()
        n757 = local write "kp"(w784) -> ()
        n758 = local write "ki"(w783) -> ()
        n759 = local write "kd"(w782) -> ()
        n760 = local write "max_step_change"(w781) -> ()
        n761 = local write "max_amplitude"(w780) -> ()
        n762 = local write "min_amplitude"(w779) -> ()
        n763 = local write "startup_cmd"(w778) -> ()
      }
    }
    n764 = local read "USER ID"() -> (w730:string)
    n765 = local write "tested by 2"(w730) -> ()
    n766 = local read "run test Calibration"() -> (w728:bool)
    n767 = disable-structure shown="Enabled" {
      disable-tunnel: [w736 w747] -> w729
      frame Disabled {
        n768 = local read "Point 1 - 0.2 mm"() -> (w746:bool)
        n769 = local read "Point 2 - 0.4 mm"() -> (w745:bool)
        n770 = local read "Point 3 - 0.6 mm"() -> (w744:bool)
        n771 = local read "Point 4 - 0.8 mm"() -> (w743:bool)
        n772 = local read "Point 5 - 1.0 mm"() -> (w742:bool)
        n773 = local read "Point 6 - 1.2 mm"() -> (w741:bool)
        n774 = And(x=w746, y=w745) -> (x .and. y?=w740:bool)
        n775 = And(x=w744, y=w743) -> (x .and. y?=w739:bool)
        n776 = And(x=w742, y=w741) -> (x .and. y?=w737:bool)
        n777 = And(x=w740, y=w739) -> (x .and. y?=w738:bool)
        n778 = And(x=w738, y=w737) -> (x .and. y?=w736:bool)
      }
      frame Enabled {
        n779 = local read "Point 5 - 1.0 mm"() -> (w747:bool)
      }
    }
    n780 = local read "START TEMP"() -> (w727:bool)
    n781 = And(x=w727, y=w728) -> (x .and. y?=w726:bool)
    n782 = case shown="True" w726 {
      frame False {
        w748 = TRUE ("PAUSE")
        n783 = call "ELAPSED TIMER VI - Calibration.vi"("RESET"=w748, "PAUSE"=w748) -> ()  [unwired: 7 in, 3 out]
      }
      frame True {
        w751 = FALSE ("PAUSE")
        n784 = call "ELAPSED TIMER VI - Calibration.vi"("TARGET"=60.0, "RESET"=w751, "PAUSE"=w751) -> ("ELAPSED INDICATION"=w749:bool)  [unwired: 6 in, 2 out]
        n785 = case shown="True" w749 {
          frame False {
          }
          frame True {
            n786 = stacked-sequence {
              frame #0 {
                n787 = local write "START TEMP"(FALSE ("START TEMP")) -> ()
              }
              frame #1 {
                n788 = Wait (ms)(milliseconds to wait=u32 1500) -> ()  [unwired: 1 out]
              }
              frame #2 {
                n789 = local write "Due Write"("VC;0") -> ()
              }
              frame #3 {
                n790 = Wait (ms)(milliseconds to wait=u32 1500) -> ()  [unwired: 1 out]
              }
              frame #4 {
                n791 = local write "Due Write"("VC;0") -> ()
              }
            }
          }
        }
      }
    }
    n792 = case shown="False" w729 {
      frame False {
        n793 = property on="Accept & Save" class="Bool (strict)"("DisabledEnum"=T19."Disabled" ("Disabled")) -> ()  [unwired: 2 in, 2 out]